vi "FlexMag - 23-03-2023.vi"() -> ()   [LabVIEW 2018] (continued)
                      frame False {
                        n9835 = local write "trns 3-4 led 3"(TRUE ("trns 1-2 led 1")) -> ()
                        n9836 = Wait (ms)(milliseconds to wait=u32 100) -> ()  [unwired: 1 out]
                      }
                      frame True {
                      }
                    }
                  }
                }
              }
              frame #9 {
                n9837 = local read "ch3-4 transfer"() -> (w15268:bool)
                n9838 = case shown="True" w15268 {
                  frame False {
                  }
                  frame True {
                    n9839 = local read "ABORT"() -> (w15269:bool)
                    n9840 = case shown="False" w15269 {
                      frame False {
                        n9841 = while {
                          i -> [w15274]
                          stop <- w15275 stop-if-true
                          n9842 = Greater Or Equal?(x=w15274, y=100) -> (x >= y?=w15272:bool)
                          n9843 = case shown="True" w15272 {
                            frame False {
                            }
                            frame True {
                              n9844 = local write "trns error"(TRUE ("TRNS error")) -> ()
                              n9845 = local write "Warning Message"("Transfer process canceled!\nCH3 TGV Control Problem" ("Warning Message")) -> ()
                            }
                          }
                          n9846 = local read "CH3_TGV_Control_DI"() -> (w15271:bool)
                          n9847 = case shown="True" w15271 {
                            tunnel: [TRUE ("CH1_Trns_BP_Left_DO") FALSE ("CH1_Trns_BP_Left_DO")] -> w15270
                            frame False {
                            }
                            frame True {
                              n9848 = Wait Until Next ms Multiple(millisecond multiple=u32 200) -> ()  [unwired: 1 out]
                              n9849 = local write "CH3_TGV_Control_DO"(FALSE ("CH1_Trns_BP_Left_DO")) -> ()
                            }
                          }
                          n9850 = local read "ch3-4 transfer"() -> (w15278:bool)
                          n9851 = local read "ABORT"() -> (w15277:bool)
                          n9852 = Not(x=w15278) -> (.not. x?=w15276:bool)
                          n9853 = Compound Arithmetic op=OR(w15270, w15277, w15276) -> (w15275:bool)
                        }
                      }
                      frame True {
                      }
                    }
                  }
                }
              }
              frame #10 {
                n9854 = local read "ch3-4 transfer"() -> (w15285:bool)
                n9855 = case shown="True" w15285 {
                  frame False {
                  }
                  frame True {
                    n9856 = local read "ABORT"() -> (w15286:bool)
                    n9857 = case shown="False" w15286 {
                      frame False {
                        n9858 = local write "trns 3-4 led 4"(TRUE ("trns 1-2 led 1")) -> ()
                        n9859 = Wait (ms)(milliseconds to wait=u32 100) -> ()  [unwired: 1 out]
                      }
                      frame True {
                      }
                    }
                  }
                }
              }
              frame #11 {
                n9860 = local read "ch3-4 transfer"() -> (w15289:bool)
                n9861 = case shown="True" w15289 {
                  frame False {
                  }
                  frame True {
                    n9862 = local read "ABORT"() -> (w15290:bool)
                    n9863 = case shown="False" w15290 {
                      frame False {
                        n9864 = while {
                          i -> [w15295]
                          stop <- w15296 stop-if-true
                          n9865 = local read "CH1_Trns_Interlock_DI"() -> (w15291:bool)
                          n9866 = Greater Or Equal?(x=w15295, y=100) -> (x >= y?=w15293:bool)
                          n9867 = case shown="True" w15293 {
                            frame False {
                            }
                            frame True {
                              n9868 = local write "Warning Message"("Transfer process canceled!\nCH1 Interlock problem" ("Warning Message")) -> ()
                              n9869 = local write "trns error"(TRUE ("TRNS error")) -> ()
                            }
                          }
                          n9870 = case shown="False" w15291 {
                            tunnel: [w15300 TRUE ("CH1_Trns_BP_Left_DO")] -> w15292
                            frame False {
                              n9871 = local read "CH1_TGV_Control_DI"() -> (w15301:bool)
                              n9872 = case shown="False" w15301 {
                                tunnel: [FALSE ("CH1_Trns_BP_Left_DO") TRUE ("CH1_Trns_BP_Left_DO")] -> w15300
                                frame False {
                                n9873 = Wait Until Next ms Multiple(millisecond multiple=u32 200) -> ()  [unwired: 1 out]
                                n9874 = local write "CH1_TGV_Control_DO"(TRUE ("CH1_Trns_BP_Left_DO")) -> ()
                                }
                                frame True {
                                }
                              }
                            }
                            frame True {
                            }
                          }
                          n9875 = local read "ch3-4 transfer"() -> (w15299:bool)
                          n9876 = local read "ABORT"() -> (w15298:bool)
                          n9877 = Not(x=w15299) -> (.not. x?=w15297:bool)
                          n9878 = Compound Arithmetic op=OR(w15292, w15298, w15297) -> (w15296:bool)
                        }
                      }
                      frame True {
                      }
                    }
                  }
                }
              }
              frame #12 {
                n9879 = local read "ch3-4 transfer"() -> (w15309:bool)
                n9880 = case shown="True" w15309 {
                  frame False {
                  }
                  frame True {
                    n9881 = local read "ABORT"() -> (w15310:bool)
                    n9882 = case shown="False" w15310 {
                      frame False {
                        w15311 = TRUE ("CH3_Right_Limit_DO")
                        n9883 = local write "trns 3-4 led 5"(TRUE ("trns 1-2 led 1")) -> ()
                        n9884 = Wait (ms)(milliseconds to wait=u32 100) -> ()  [unwired: 1 out]
                        n9885 = local write "CH3_Right_Limit_DO"(w15311) -> ()
                        n9886 = local write "CH3_Right_Slow_DO"(w15311) -> ()
                        n9887 = local write "CH3_Left_Slow_DO"(w15311) -> ()
                        n9888 = local write "CH3_Left_Limit_DO"(w15311) -> ()
                      }
                      frame True {
                      }
                    }
                  }
                }
              }
              frame #13 {
                n9889 = local read "ch3-4 transfer"() -> (w15314:bool)
                n9890 = case shown="True" w15314 {
                  frame False {
                  }
                  frame True {
                    n9891 = local read "ABORT"() -> (w15315:bool)
                    n9892 = case shown="False" w15315 {
                      frame False {
                        n9893 = while {
                          i -> [w15320]
                          stop <- w15321 stop-if-true
                          n9894 = local read "CH2_Trns_Interlock_DI"() -> (w15316:bool)
                          n9895 = Greater Or Equal?(x=w15320, y=100) -> (x >= y?=w15318:bool)
                          n9896 = case shown="True" w15318 {
                            frame False {
                            }
                            frame True {
                              n9897 = local write "Warning Message"("Transfer process canceled!\nCH2 Interlock problem" ("Warning Message")) -> ()
                              n9898 = local write "trns error"(TRUE ("TRNS error")) -> ()
                            }
                          }
                          n9899 = case shown="False" w15316 {
                            tunnel: [w15325 TRUE ("CH1_Trns_BP_Left_DO")] -> w15317
                            frame False {
                              n9900 = local read "CH2_TGV_Control_DI"() -> (w15326:bool)
                              n9901 = case shown="False" w15326 {
                                tunnel: [FALSE ("CH1_Trns_BP_Left_DO") TRUE ("CH1_Trns_BP_Left_DO")] -> w15325
                                frame False {
                                n9902 = Wait Until Next ms Multiple(millisecond multiple=u32 200) -> ()  [unwired: 1 out]
                                n9903 = local write "CH2_TGV_Control_DO"(TRUE ("CH1_Trns_BP_Left_DO")) -> ()
                                }
                                frame True {
                                }
                              }
                            }
                            frame True {
                            }
                          }
                          n9904 = local read "ch3-4 transfer"() -> (w15324:bool)
                          n9905 = local read "ABORT"() -> (w15323:bool)
                          n9906 = Not(x=w15324) -> (.not. x?=w15322:bool)
                          n9907 = Compound Arithmetic op=OR(w15317, w15323, w15322) -> (w15321:bool)
                        }
                      }
                      frame True {
                      }
                    }
                  }
                }
              }
              frame #14 {
                n9908 = local read "ch3-4 transfer"() -> (w15334:bool)
                n9909 = case shown="True" w15334 {
                  frame False {
                  }
                  frame True {
                    n9910 = local read "ABORT"() -> (w15335:bool)
                    n9911 = case shown="False" w15335 {
                      frame False {
                        n9912 = local write "trns 3-4 led 6"(TRUE ("trns 1-2 led 1")) -> ()
                        n9913 = Wait (ms)(milliseconds to wait=u32 100) -> ()  [unwired: 1 out]
                      }
                      frame True {
                      }
                    }
                  }
                }
              }
              frame #15 {
                n9914 = local read "ch3-4 transfer"() -> (w15338:bool)
                n9915 = case shown="True" w15338 {
                  frame False {
                  }
                  frame True {
                    n9916 = local read "ABORT"() -> (w15339:bool)
                    n9917 = case shown="False" w15339 {
                      frame False {
                        n9918 = while {
                          i -> [w15344]
                          stop <- w15345 stop-if-true
                          n9919 = local read "CH4_Trns_Interlock_DI"() -> (w15340:bool)
                          n9920 = Greater Or Equal?(x=w15344, y=100) -> (x >= y?=w15342:bool)
                          n9921 = case shown="True" w15342 {
                            frame False {
                            }
                            frame True {
                              n9922 = local write "Warning Message"("Transfer process canceled!\nCH4 Interlock problem" ("Warning Message")) -> ()
                              n9923 = local write "trns error"(TRUE ("TRNS error")) -> ()
                            }
                          }
                          n9924 = case shown="False" w15340 {
                            tunnel: [w15349 TRUE ("CH1_Trns_BP_Left_DO")] -> w15341
                            frame False {
                              n9925 = local read "CH4_TGV_Control_DI"() -> (w15350:bool)
                              n9926 = case shown="False" w15350 {
                                tunnel: [FALSE ("CH1_Trns_BP_Left_DO") TRUE ("CH1_Trns_BP_Left_DO")] -> w15349
                                frame False {
                                n9927 = Wait Until Next ms Multiple(millisecond multiple=u32 200) -> ()  [unwired: 1 out]
                                n9928 = local write "CH4_TGV_Control_DO"(TRUE ("CH1_Trns_BP_Left_DO")) -> ()
                                }
                                frame True {
                                }
                              }
                            }
                            frame True {
                            }
                          }
                          n9929 = local read "ch3-4 transfer"() -> (w15348:bool)
                          n9930 = local read "ABORT"() -> (w15347:bool)
                          n9931 = Not(x=w15348) -> (.not. x?=w15346:bool)
                          n9932 = Compound Arithmetic op=OR(w15341, w15347, w15346) -> (w15345:bool)
                        }
                      }
                      frame True {
                      }
                    }
                  }
                }
              }
              frame #16 {
                n9933 = local read "ch3-4 transfer"() -> (w15358:bool)
                n9934 = case shown="True" w15358 {
                  frame False {
                  }
                  frame True {
                    n9935 = local read "ABORT"() -> (w15359:bool)
                    n9936 = case shown="False" w15359 {
                      frame False {
                        n9937 = local write "trns 3-4 led 7"(TRUE ("trns 1-2 led 1")) -> ()
                        n9938 = Wait (ms)(milliseconds to wait=u32 100) -> ()  [unwired: 1 out]
                      }
                      frame True {
                      }
                    }
                  }
                }
              }
              frame #17 {
                n9939 = local read "ch3-4 transfer"() -> (w15362:bool)
                n9940 = case shown="True" w15362 {
                  frame False {
                  }
                  frame True {
                    n9941 = local read "ABORT"() -> (w15363:bool)
                    n9942 = case shown="False" w15363 {
                      frame False {
                        n9943 = while {
                          i -> [w15367]
                          stop <- w15368 stop-if-true
                          n9944 = Greater Or Equal?(x=w15367, y=100) -> (x >= y?=w15365:bool)
                          n9945 = case shown="True" w15365 {
                            frame False {
                            }
                            frame True {
                              n9946 = local write "Warning Message"("Transfer process canceled!\nRight Slow Sensor problem" ("Warning Message")) -> ()
                              n9947 = local write "trns error"(TRUE ("TRNS error")) -> ()
                            }
                          }
                          n9948 = disable-structure shown="Enabled" {
                            disable-tunnel: [w15373 w15378] -> w15364
                            frame Disabled {
                              n9949 = local read "Cnt_Right_Slow DI"() -> (w15372:bool)
                              n9950 = case shown="False" w15372 {
                                tunnel: [FALSE ("CH1_Trns_BP_Left_DO") TRUE ("CH1_Trns_BP_Left_DO")] -> w15373
                                frame False {
                                n9951 = Wait Until Next ms Multiple(millisecond multiple=u32 200) -> ()  [unwired: 1 out]
                                n9952 = local write "Cnt_Right_Slow DO"(TRUE ("CH1_Trns_BP_Left_DO")) -> ()
                                }
                                frame True {
                                }
                              }
                            }
                            frame Enabled {
                              n9953 = local read "CH3_Right_Slow_DI"() -> (w15379:bool)
                              n9954 = case shown="True" w15379 {
                                tunnel: [TRUE FALSE] -> w15378
                                frame False {
                                }
                                frame True {
                                n9955 = Wait Until Next ms Multiple(millisecond multiple=u32 200) -> ()  [unwired: 1 out]
                                n9956 = local write "CH3_Right_Slow_DO"(TRUE ("CH2_Right_Limit_DO")) -> ()
                                }
                              }
                            }
                          }
                          n9957 = local read "ch3-4 transfer"() -> (w15371:bool)
                          n9958 = local read "ABORT"() -> (w15370:bool)
                          n9959 = Not(x=w15371) -> (.not. x?=w15369:bool)
                          n9960 = Compound Arithmetic op=OR(w15364, w15370, w15369) -> (w15368:bool)
                        }
                      }
                      frame True {
                      }
                    }
                  }
                }
              }
              frame #18 {
                n9961 = local read "ch3-4 transfer"() -> (w15386:bool)
                n9962 = case shown="True" w15386 {
                  frame False {
                  }
                  frame True {
                    n9963 = local read "ABORT"() -> (w15387:bool)
                    n9964 = case shown="False" w15387 {
                      frame False {
                        n9965 = local write "trns 3-4 led 8"(TRUE ("trns 1-2 led 1")) -> ()
                        n9966 = Wait (ms)(milliseconds to wait=u32 100) -> ()  [unwired: 1 out]
                      }
                      frame True {
                      }
                    }
                  }
                }
              }
              frame #19 {
                n9967 = local read "ch3-4 transfer"() -> (w15390:bool)
                n9968 = case shown="True" w15390 {
                  frame False {
                  }
                  frame True {
                    n9969 = local read "ABORT"() -> (w15391:bool)
                    n9970 = case shown="False" w15391 {
                      frame False {
                        n9971 = while {
                          i -> [w15395]
                          stop <- w15396 stop-if-true
                          n9972 = Greater Or Equal?(x=w15395, y=100) -> (x >= y?=w15393:bool)
                          n9973 = case shown="True" w15393 {
                            frame False {
                            }
                            frame True {
                              n9974 = local write "Warning Message"("Transfer process canceled!\nRight Limit Sensor problem" ("Warning Message")) -> ()
                              n9975 = local write "trns error"(TRUE ("TRNS error")) -> ()
                            }
                          }
                          n9976 = disable-structure shown="Enabled" {
                            disable-tunnel: [w15401 w15406] -> w15392
                            frame Disabled {
                              n9977 = local read "Cnt_Right_Limit DI"() -> (w15400:bool)
                              n9978 = case shown="False" w15400 {
                                tunnel: [FALSE ("CH1_Trns_BP_Left_DO") TRUE ("CH1_Trns_BP_Left_DO")] -> w15401
                                frame False {
                                n9979 = Wait Until Next ms Multiple(millisecond multiple=u32 200) -> ()  [unwired: 1 out]
                                n9980 = local write "Cnt_Right_Limit DO"(TRUE ("CH1_Trns_BP_Left_DO")) -> ()
                                }
                                frame True {
                                }
                              }
                            }
                            frame Enabled {
                              n9981 = local read "CH3_Right_Limit_DI"() -> (w15407:bool)
                              n9982 = case shown="True" w15407 {
                                tunnel: [TRUE FALSE] -> w15406
                                frame False {
                                }
                                frame True {
                                n9983 = Wait Until Next ms Multiple(millisecond multiple=u32 200) -> ()  [unwired: 1 out]
                                n9984 = local write "CH3_Right_Limit_DO"(TRUE ("CH2_Right_Limit_DO")) -> ()
                                }
                              }
                            }
                          }
                          n9985 = local read "ch3-4 transfer"() -> (w15399:bool)
                          n9986 = local read "ABORT"() -> (w15398:bool)
                          n9987 = Not(x=w15399) -> (.not. x?=w15397:bool)
                          n9988 = Compound Arithmetic op=OR(w15392, w15398, w15397) -> (w15396:bool)
                        }
                      }
                      frame True {
                      }
                    }
                  }
                }
              }
              frame #20 {
                n9989 = local read "ch3-4 transfer"() -> (w15414:bool)
                n9990 = case shown="True" w15414 {
                  frame False {
                  }
                  frame True {
                    n9991 = local read "ABORT"() -> (w15415:bool)
                    n9992 = case shown="False" w15415 {
                      frame False {
                        n9993 = local write "trns 3-4 led 9"(TRUE ("trns 1-2 led 1")) -> ()
                        n9994 = Wait (ms)(milliseconds to wait=u32 100) -> ()  [unwired: 1 out]
                      }
                      frame True {
                      }
                    }
                  }
                }
              }
              frame #21 {
                n9995 = local read "ch3-4 transfer"() -> (w15418:bool)
                n9996 = case shown="True" w15418 {
                  frame False {
                  }
                  frame True {
                    n9997 = local read "ABORT"() -> (w15419:bool)
                    n9998 = case shown="False" w15419 {
                      frame False {
                        n9999 = while {
                          i -> [w15423]
                          stop <- w15424 stop-if-true
                          n10000 = Greater Or Equal?(x=w15423, y=100) -> (x >= y?=w15421:bool)
                          n10001 = case shown="True" w15421 {
                            frame False {
                            }
                            frame True {
                              n10002 = local write "Warning Message"("Transfer process canceled!\nLeft Slow Sensor problem" ("Warning Message")) -> ()
                              n10003 = local write "trns error"(TRUE ("TRNS error")) -> ()
                            }
                          }
                          n10004 = disable-structure shown="Enabled" {
                            disable-tunnel: [w15429 w15434] -> w15420
                            frame Disabled {
                              n10005 = local read "Cnt_Left_Slow DI"() -> (w15428:bool)
                              n10006 = case shown="False" w15428 {
                                tunnel: [FALSE ("CH1_Trns_BP_Left_DO") TRUE ("CH1_Trns_BP_Left_DO")] -> w15429
                                frame False {
                                n10007 = Wait Until Next ms Multiple(millisecond multiple=u32 200) -> ()  [unwired: 1 out]
                                n10008 = local write "Cnt_Left_Slow DO"(TRUE ("CH1_Trns_BP_Left_DO")) -> ()
                                }
                                frame True {
                                }
                              }
                            }
                            frame Enabled {
                              n10009 = local read "CH3_Left_Slow_DI"() -> (w15435:bool)
                              n10010 = case shown="True" w15435 {
                                tunnel: [TRUE FALSE] -> w15434
                                frame False {
                                }
                                frame True {
                                n10011 = Wait Until Next ms Multiple(millisecond multiple=u32 200) -> ()  [unwired: 1 out]
                                n10012 = local write "CH3_Left_Slow_DO"(TRUE ("CH2_Right_Limit_DO")) -> ()
                                }
                              }
                            }
                          }
                          n10013 = local read "ch3-4 transfer"() -> (w15427:bool)
                          n10014 = local read "ABORT"() -> (w15426:bool)
                          n10015 = Not(x=w15427) -> (.not. x?=w15425:bool)
                          n10016 = Compound Arithmetic op=OR(w15420, w15426, w15425) -> (w15424:bool)
                        }
                      }
                      frame True {
                      }
                    }
                  }
                }
              }
              frame #22 {
                n10017 = local read "ch3-4 transfer"() -> (w15442:bool)
                n10018 = case shown="True" w15442 {
                  frame False {
                  }
                  frame True {
                    n10019 = local read "ABORT"() -> (w15443:bool)
                    n10020 = case shown="False" w15443 {
                      frame False {
                        n10021 = local write "trns 3-4 led 10"(TRUE ("trns 1-2 led 1")) -> ()
                        n10022 = Wait (ms)(milliseconds to wait=u32 100) -> ()  [unwired: 1 out]
                      }
                      frame True {
                      }
                    }
                  }
                }
              }
              frame #23 {
                n10023 = local read "ch3-4 transfer"() -> (w15446:bool)
                n10024 = case shown="True" w15446 {
                  frame False {
                  }
                  frame True {
                    n10025 = local read "ABORT"() -> (w15447:bool)
                    n10026 = case shown="False" w15447 {
                      frame False {
                        n10027 = while {
                          i -> [w15451]
                          stop <- w15452 stop-if-true
                          n10028 = Greater Or Equal?(x=w15451, y=100) -> (x >= y?=w15449:bool)
                          n10029 = case shown="True" w15449 {
                            frame False {
                            }
                            frame True {
                              n10030 = local write "Warning Message"("Transfer process canceled!\nLeft Limit Sensor problem" ("Warning Message")) -> ()
                              n10031 = local write "trns error"(TRUE ("TRNS error")) -> ()
                            }
                          }
                          n10032 = disable-structure shown="Enabled" {
                            disable-tunnel: [w15457 w15462] -> w15448
                            frame Disabled {
                              n10033 = local read "Cnt_Left_Limit DI"() -> (w15456:bool)
                              n10034 = case shown="False" w15456 {
                                tunnel: [FALSE ("CH1_Trns_BP_Left_DO") TRUE ("CH1_Trns_BP_Left_DO")] -> w15457
                                frame False {
                                n10035 = Wait Until Next ms Multiple(millisecond multiple=u32 200) -> ()  [unwired: 1 out]
                                n10036 = local write "Cnt_Left_Limit DO"(TRUE ("CH1_Trns_BP_Left_DO")) -> ()
                                }
                                frame True {
                                }
                              }
                            }
                            frame Enabled {
                              n10037 = local read "CH3_Left_Limit_DI"() -> (w15463:bool)
                              n10038 = case shown="True" w15463 {
                                tunnel: [TRUE FALSE] -> w15462
                                frame False {
                                }
                                frame True {
                                n10039 = Wait Until Next ms Multiple(millisecond multiple=u32 200) -> ()  [unwired: 1 out]
                                n10040 = local write "CH3_Left_Limit_DO"(TRUE ("CH2_Right_Limit_DO")) -> ()
                                }
                              }
                            }
                          }
                          n10041 = local read "ch3-4 transfer"() -> (w15455:bool)
                          n10042 = local read "ABORT"() -> (w15454:bool)
                          n10043 = Not(x=w15455) -> (.not. x?=w15453:bool)
                          n10044 = Compound Arithmetic op=OR(w15448, w15454, w15453) -> (w15452:bool)
                        }
                      }
                      frame True {
                      }
                    }
                  }
                }
              }
              frame #24 {
                n10045 = local read "ch3-4 transfer"() -> (w15470:bool)
                n10046 = case shown="True" w15470 {
                  frame False {
                  }
                  frame True {
                    n10047 = local read "ABORT"() -> (w15471:bool)
                    n10048 = case shown="False" w15471 {
                      frame False {
                        n10049 = local write "trns 3-4 led 11"(TRUE ("trns 1-2 led 1")) -> ()
                        n10050 = Wait (ms)(milliseconds to wait=u32 100) -> ()  [unwired: 1 out]
                      }
                      frame True {
                      }
                    }
                  }
                }
              }
              frame #25 {
                n10051 = local read "ch3-4 transfer"() -> (w15474:bool)
                n10052 = case shown="True" w15474 {
                  frame False {
                  }
                  frame True {
                    n10053 = local read "ABORT"() -> (w15475:bool)
                    n10054 = case shown="False" w15475 {
                      frame False {
                        w15476 = FALSE ("CH4_SRV1_Piston_For_DO")
                        n10055 = local write "CH4_Left_Limit_DO"(w15476) -> ()
                        n10056 = local write "CH4_Left_Slow_DO"(w15476) -> ()
                        n10057 = Wait (ms)(milliseconds to wait=u32 2000) -> ()  [unwired: 1 out]
                      }
                      frame True {
                      }
                    }
                  }
                }
              }
              frame #26 {
                n10058 = local read "ch3-4 transfer"() -> (w15478:bool)
                n10059 = case shown="True" w15478 {
                  frame False {
                  }
                  frame True {
                    n10060 = local read "ABORT"() -> (w15479:bool)
                    n10061 = case shown="False" w15479 {
                      frame False {
                        n10062 = while {
                          i -> [w15484]
                          stop <- w15485 stop-if-true
                          n10063 = Greater Or Equal?(x=w15484, y=100) -> (x >= y?=w15482:bool)
                          n10064 = case shown="True" w15482 {
                            frame False {
                            }
                            frame True {
                              n10065 = local write "Warning Message"("Transfer process canceled!\nCassette Servo Direction problem" ("Warning Message")) -> ()
                              n10066 = local write "trns error"(TRUE ("TRNS error")) -> ()
                            }
                          }
                          n10067 = local read "Casette_Servo_Left_Direction DI"() -> (w15480:bool)
                          n10068 = case shown="False" w15480 {
                            tunnel: [FALSE ("CH1_Trns_BP_Left_DO") TRUE ("CH1_Trns_BP_Left_DO")] -> w15481
                            frame False {
                              n10069 = local write "Casette_Servo_Left_Direction DO"(TRUE ("CH1_Trns_BP_Left_DO")) -> ()
                              n10070 = Wait Until Next ms Multiple(millisecond multiple=u32 200) -> ()  [unwired: 1 out]
                            }
                            frame True {
                            }
                          }
                          n10071 = local read "ch3-4 transfer"() -> (w15488:bool)
                          n10072 = local read "ABORT"() -> (w15487:bool)
                          n10073 = Not(x=w15488) -> (.not. x?=w15486:bool)
                          n10074 = Compound Arithmetic op=OR(w15481, w15487, w15486) -> (w15485:bool)
                        }
                      }
                      frame True {
                      }
                    }
                  }
                }
              }
              frame #27 {
                n10075 = local read "ch3-4 transfer"() -> (w15495:bool)
                n10076 = case shown="True" w15495 {
                  frame False {
                  }
                  frame True {
                    n10077 = local read "ABORT"() -> (w15496:bool)
                    n10078 = case shown="False" w15496 {
                      frame False {
                        n10079 = local write "trns 3-4 led 12"(TRUE ("trns 1-2 led 1")) -> ()
                        n10080 = Wait (ms)(milliseconds to wait=u32 100) -> ()  [unwired: 1 out]
                      }
                      frame True {
                      }
                    }
                  }
                }
              }
              frame #28 {
                n10081 = local read "ch3-4 transfer"() -> (w15499:bool)
                n10082 = case shown="True" w15499 {
                  frame False {
                  }
                  frame True {
                    n10083 = local read "ABORT"() -> (w15500:bool)
                    n10084 = case shown="False" w15500 {
                      frame False {
                        n10085 = stacked-sequence {
                          frame #0 {
                            n10086 = local read "Cst_Speed_High"() -> (w15501:dbl)
                            n10087 = Wait (ms)(milliseconds to wait=u32 100) -> ()  [unwired: 1 out]
                            n10088 = local write "Cassette_Servo_Speed AO"(w15501) -> ()
                          }
                          frame #1 {
                            n10089 = Wait (ms)(milliseconds to wait=u32 200) -> ()  [unwired: 1 out]
                          }
                          frame #2 {
                            n10090 = local write "Cassette_Servo_Speed Set"(TRUE ("Cassette_Servo_Speed Set")) -> ()
                          }
                          frame #3 {
                            n10091 = Wait (ms)(milliseconds to wait=u32 300) -> ()  [unwired: 1 out]
                          }
                        }
                      }
                      frame True {
                      }
                    }
                  }
                }
              }
              frame #29 {
                n10092 = local read "ch3-4 transfer"() -> (w15506:bool)
                n10093 = case shown="True" w15506 {
                  frame False {
                  }
                  frame True {
                    n10094 = local read "ABORT"() -> (w15507:bool)
                    n10095 = case shown="False" w15507 {
                      frame False {
                        n10096 = local write "trns 3-4 led 13"(TRUE ("trns 1-2 led 1")) -> ()
                        n10097 = Wait (ms)(milliseconds to wait=u32 100) -> ()  [unwired: 1 out]
                      }
                      frame True {
                      }
                    }
                  }
                }
              }
              frame #30 {
                n10098 = local read "ch3-4 transfer"() -> (w15510:bool)
                n10099 = case shown="True" w15510 {
                  frame False {
                  }
                  frame True {
                    n10100 = local read "ABORT"() -> (w15511:bool)
                    n10101 = case shown="False" w15511 {
                      frame False {
                        n10102 = while {
                          i -> [w15516]
                          stop <- w15517 stop-if-true
                          n10103 = Greater Or Equal?(x=w15516, y=100) -> (x >= y?=w15514:bool)
                          n10104 = case shown="True" w15514 {
                            frame False {
                            }
                            frame True {
                              n10105 = local write "Warning Message"("Transfer process canceled!\nCassette Servo Start problem" ("Warning Message")) -> ()
                              n10106 = local write "trns error"(TRUE ("TRNS error")) -> ()
                            }
                          }
                          n10107 = local read "Casette_Servo_Start/Stop DI"() -> (w15512:bool)
                          n10108 = case shown="False" w15512 {
                            tunnel: [FALSE ("CH1_Trns_BP_Left_DO") TRUE ("CH1_Trns_BP_Left_DO")] -> w15513
                            frame False {
                              n10109 = local write "Casette_Servo_Start/Stop DO"(TRUE ("CH1_Trns_BP_Left_DO")) -> ()
                              n10110 = Wait Until Next ms Multiple(millisecond multiple=u32 200) -> ()  [unwired: 1 out]
                            }
                            frame True {
                            }
                          }
                          n10111 = local read "ch3-4 transfer"() -> (w15520:bool)
                          n10112 = local read "ABORT"() -> (w15519:bool)
                          n10113 = Not(x=w15520) -> (.not. x?=w15518:bool)
                          n10114 = Compound Arithmetic op=OR(w15513, w15519, w15518) -> (w15517:bool)
                        }
                      }
                      frame True {
                      }
                    }
                  }
                }
              }
              frame #31 {
                n10115 = local read "ch3-4 transfer"() -> (w15527:bool)
                n10116 = case shown="True" w15527 {
                  frame False {
                  }
                  frame True {
                    n10117 = local read "ABORT"() -> (w15528:bool)
                    n10118 = case shown="False" w15528 {
                      frame False {
                        n10119 = local write "trns 3-4 led 14"(TRUE ("trns 1-2 led 1")) -> ()
                        n10120 = Wait (ms)(milliseconds to wait=u32 100) -> ()  [unwired: 1 out]
                      }
                      frame True {
                      }
                    }
                  }
                }
              }
              frame #32 {
                n10121 = local read "ch3-4 transfer"() -> (w15531:bool)
                n10122 = case shown="True" w15531 {
                  frame False {
                  }
                  frame True {
                    n10123 = local read "ABORT"() -> (w15532:bool)
                    n10124 = case shown="False" w15532 {
                      frame False {
                        n10125 = disable-structure shown="Disabled" {
                          frame Disabled {
                            n10126 = stacked-sequence {
                              frame #0 {
                                n10127 = while {
                                i -> [w15539]
                                stop <- w15540 stop-if-true
                                n10128 = Greater Or Equal?(x=w15539, y=1500) -> (x >= y?=w15537:bool)
                                n10129 = case shown="True" w15537 {
                                frame False {
                                }
                                frame True {
                                n10130 = local write "Warning Message"("Transfer process canceled!\nCounter problem" ("Warning Message")) -> ()
                                n10131 = local write "trns error"(TRUE ("TRNS error")) -> ()
                                }
                                }
                                n10132 = local read "Counter Read Data"() -> (w15535:i16)
                                n10133 = Greater Or Equal?(x=w15535, y=i16 5820) -> (x >= y?=w15533:bool)
                                n10134 = case shown="True" w15533 {
                                tunnel: [FALSE ("CH1_Trns_BP_Left_DO") TRUE ("CH1_Trns_BP_Left_DO")] -> w15536
                                frame False {
                                n10135 = Wait Until Next ms Multiple(millisecond multiple=u32 200) -> ()  [unwired: 1 out]
                                }
                                frame True {
                                }
                                }
                                n10136 = local read "ch3-4 transfer"() -> (w15543:bool)
                                n10137 = local read "ABORT"() -> (w15542:bool)
                                n10138 = Not(x=w15543) -> (.not. x?=w15541:bool)
                                n10139 = Compound Arithmetic op=OR(w15536, w15542, w15541) -> (w15540:bool)
                                }
                              }
                              frame #1 {
                                n10140 = while {
                                i -> [w15553]
                                stop <- w15554 stop-if-true
                                n10141 = Greater Or Equal?(x=w15553, y=100) -> (x >= y?=w15551:bool)
                                n10142 = case shown="True" w15551 {
                                frame False {
                                }
                                frame True {
                                n10143 = local write "Warning Message"("Transfer process canceled!\nLeft Slow Sensor problem" ("Warning Message")) -> ()
                                n10144 = local write "trns error"(TRUE ("TRNS error")) -> ()
                                }
                                }
                                n10145 = local read "Cnt_Left_Slow DI"() -> (w15549:bool)
                                n10146 = case shown="True" w15549 {
                                tunnel: [TRUE ("CH1_Trns_BP_Left_DO") FALSE ("CH1_Trns_BP_Left_DO")] -> w15550
                                frame False {
                                }
                                frame True {
                                n10147 = Wait Until Next ms Multiple(millisecond multiple=u32 200) -> ()  [unwired: 1 out]
                                n10148 = local write "Cnt_Left_Slow DO"(FALSE ("TRNS error")) -> ()
                                }
                                }
                                n10149 = local read "ch3-4 transfer"() -> (w15557:bool)
                                n10150 = local read "ABORT"() -> (w15556:bool)
                                n10151 = Not(x=w15557) -> (.not. x?=w15555:bool)
                                n10152 = Compound Arithmetic op=OR(w15550, w15556, w15555) -> (w15554:bool)
                                }
                              }
                              frame #2 {
                                n10153 = while {
                                i -> [w15568]
                                stop <- w15569 stop-if-true
                                n10154 = Greater Or Equal?(x=w15568, y=100) -> (x >= y?=w15566:bool)
                                n10155 = case shown="True" w15566 {
                                frame False {
                                }
                                frame True {
                                n10156 = local write "Warning Message"("Transfer process canceled!\nLeft Limit Sensor problem" ("Warning Message")) -> ()
                                n10157 = local write "trns error"(TRUE ("TRNS error")) -> ()
                                }
                                }
                                n10158 = local read "Cnt_Left_Limit DI"() -> (w15564:bool)
                                n10159 = case shown="True" w15564 {
                                tunnel: [TRUE ("CH1_Trns_BP_Left_DO") FALSE ("CH1_Trns_BP_Left_DO")] -> w15565
                                frame False {
                                }
                                frame True {
                                n10160 = Wait Until Next ms Multiple(millisecond multiple=u32 200) -> ()  [unwired: 1 out]
                                n10161 = local write "Cnt_Left_Limit DO"(FALSE ("TRNS error")) -> ()
                                }
                                }
                                n10162 = local read "ch3-4 transfer"() -> (w15572:bool)
                                n10163 = local read "ABORT"() -> (w15571:bool)
                                n10164 = Not(x=w15572) -> (.not. x?=w15570:bool)
                                n10165 = Compound Arithmetic op=OR(w15565, w15571, w15570) -> (w15569:bool)
                                }
                              }
                            }
                          }
                          frame Enabled {
                          }
                        }
                      }
                      frame True {
                      }
                    }
                  }
                }
              }
              frame #33 {
                n10166 = local read "ch3-4 transfer"() -> (w15579:bool)
                n10167 = case shown="True" w15579 {
                  frame False {
                  }
                  frame True {
                    n10168 = local read "ABORT"() -> (w15580:bool)
                    n10169 = case shown="False" w15580 {
                      frame False {
                        n10170 = local write "trns 3-4 led 15"(TRUE ("trns 1-2 led 1")) -> ()
                        n10171 = Wait (ms)(milliseconds to wait=u32 100) -> ()  [unwired: 1 out]
                      }
                      frame True {
                      }
                    }
                  }
                }
              }
              frame #34 {
                n10172 = local read "ch3-4 transfer"() -> (w15583:bool)
                n10173 = case shown="True" w15583 {
                  frame False {
                  }
                  frame True {
                    n10174 = local read "ABORT"() -> (w15584:bool)
                    n10175 = case shown="False" w15584 {
                      frame False {
                        n10176 = stacked-sequence {
                          frame #0 {
                            n10177 = while {
                              i -> [w15589]
                              stop <- w15590 stop-if-true
                              n10178 = Greater Or Equal?(x=w15589, y=1500) -> (x >= y?=w15587:bool)
                              n10179 = case shown="True" w15587 {
                                frame False {
                                }
                                frame True {
                                n10180 = local write "Warning Message"("Transfer process canceled!\nCH4 Left Slow Sensor problem" ("Warning Message")) -> ()
                                n10181 = local write "trns error"(TRUE ("TRNS error")) -> ()
                                }
                              }
                              n10182 = local read "CH4_Left_Slow_DI"() -> (w15585:bool)
                              n10183 = case shown="True" w15585 {
                                tunnel: [FALSE ("CH1_Trns_BP_Left_DO") TRUE ("CH1_Trns_BP_Left_DO")] -> w15586
                                frame False {
                                n10184 = Wait Until Next ms Multiple(millisecond multiple=u32 200) -> ()  [unwired: 1 out]
                                }
                                frame True {
                                }
                              }
                              n10185 = local read "ch3-4 transfer"() -> (w15593:bool)
                              n10186 = local read "ABORT"() -> (w15592:bool)
                              n10187 = Not(x=w15593) -> (.not. x?=w15591:bool)
                              n10188 = Compound Arithmetic op=OR(w15586, w15592, w15591) -> (w15590:bool)
                            }
                          }
                          frame #1 {
                            n10189 = flat-sequence {
                              frame #0 {
                                n10190 = local read "Cst_Speed_Low"() -> (w15599:dbl)
                                n10191 = local write "Cassette_Servo_Speed AO"(w15599) -> ()
                                n10192 = Wait (ms)(milliseconds to wait=u32 100) -> ()  [unwired: 1 out]
                              }
                              frame #1 {
                                n10193 = local write "Cassette_Servo_Speed Set"(TRUE ("Cassette_Servo_Speed Set")) -> ()
                              }
                              frame #2 {
                                n10194 = Wait (ms)(milliseconds to wait=u32 100) -> ()  [unwired: 1 out]
                              }
                            }
                          }
                          frame #2 {
                            n10195 = while {
                              i -> [w15606]
                              stop <- w15607 stop-if-true
                              n10196 = Greater Or Equal?(x=w15606, y=100) -> (x >= y?=w15604:bool)
                              n10197 = case shown="True" w15604 {
                                frame False {
                                }
                                frame True {
                                n10198 = local write "Warning Message"("Transfer process canceled!\nLeft Slow Sensor problem" ("Warning Message")) -> ()
                                n10199 = local write "trns error"(TRUE ("TRNS error")) -> ()
                                }
                              }
                              n10200 = disable-structure shown="Enabled" {
                                disable-tunnel: [w15612 w15617] -> w15603
                                frame Disabled {
                                n10201 = local read "Cnt_Left_Slow DI"() -> (w15611:bool)
                                n10202 = case shown="False" w15611 {
                                tunnel: [FALSE ("CH1_Trns_BP_Left_DO") TRUE ("CH1_Trns_BP_Left_DO")] -> w15612
                                frame False {
                                n10203 = Wait Until Next ms Multiple(millisecond multiple=u32 200) -> ()  [unwired: 1 out]
                                n10204 = local write "Cnt_Left_Slow DO"(TRUE ("TRNS error")) -> ()
                                }
                                frame True {
                                }
                                }
                                }
                                frame Enabled {
                                n10205 = local read "CH4_Left_Slow_DI"() -> (w15618:bool)
                                n10206 = case shown="True" w15618 {
                                tunnel: [TRUE FALSE] -> w15617
                                frame False {
                                }
                                frame True {
                                n10207 = Wait Until Next ms Multiple(millisecond multiple=u32 200) -> ()  [unwired: 1 out]
                                n10208 = local write "CH4_Left_Slow_DO"(TRUE ("CH2_Right_Limit_DO")) -> ()
                                }
                                }
                                }
                              }
                              n10209 = local read "ch3-4 transfer"() -> (w15610:bool)
                              n10210 = local read "ABORT"() -> (w15609:bool)
                              n10211 = Not(x=w15610) -> (.not. x?=w15608:bool)
                              n10212 = Compound Arithmetic op=OR(w15603, w15609, w15608) -> (w15607:bool)
                            }
                          }
                        }
                      }
                      frame True {
                      }
                    }
                  }
                }
              }
              frame #35 {
                n10213 = local read "ch3-4 transfer"() -> (w15625:bool)
                n10214 = case shown="True" w15625 {
                  frame False {
                  }
                  frame True {
                    n10215 = local read "ABORT"() -> (w15626:bool)
                    n10216 = case shown="False" w15626 {
                      frame False {
                        n10217 = local write "trns 3-4 led 16"(TRUE ("trns 1-2 led 1")) -> ()
                        n10218 = Wait (ms)(milliseconds to wait=u32 100) -> ()  [unwired: 1 out]
                      }
                      frame True {
                      }
                    }
                  }
                }
              }
              frame #36 {
                n10219 = local read "ch3-4 transfer"() -> (w15629:bool)
                n10220 = case shown="True" w15629 {
                  frame False {
                  }
                  frame True {
                    n10221 = local read "ABORT"() -> (w15630:bool)
                    n10222 = case shown="False" w15630 {
                      frame False {
                        n10223 = stacked-sequence {
                          frame #0 {
                            n10224 = while {
                              i -> [w15635]
                              stop <- w15636 stop-if-true
                              n10225 = Greater Or Equal?(x=w15635, y=600) -> (x >= y?=w15633:bool)
                              n10226 = case shown="True" w15633 {
                                frame False {
                                }
                                frame True {
                                n10227 = local write "Warning Message"("Transfer process canceled!\nCH4 Left Limit Sensor problem" ("Warning Message")) -> ()
                                n10228 = local write "trns error"(TRUE ("TRNS error")) -> ()
                                }
                              }
                              n10229 = local read "CH4_Left_Limit_DI"() -> (w15631:bool)
                              n10230 = case shown="True" w15631 {
                                tunnel: [FALSE ("CH1_Trns_BP_Left_DO") TRUE ("CH1_Trns_BP_Left_DO")] -> w15632
                                frame False {
                                n10231 = Wait Until Next ms Multiple(millisecond multiple=u32 200) -> ()  [unwired: 1 out]
                                }
                                frame True {
                                }
                              }
                              n10232 = local read "ch3-4 transfer"() -> (w15639:bool)
                              n10233 = local read "ABORT"() -> (w15638:bool)
                              n10234 = Not(x=w15639) -> (.not. x?=w15637:bool)
                              n10235 = Compound Arithmetic op=OR(w15632, w15638, w15637) -> (w15636:bool)
                            }
                          }
                          frame #1 {
                            n10236 = while {
                              i -> [w15649]
                              stop <- w15650 stop-if-true
                              n10237 = Greater Or Equal?(x=w15649, y=100) -> (x >= y?=w15647:bool)
                              n10238 = case shown="True" w15647 {
                                frame False {
                                }
                                frame True {
                                n10239 = local write "Warning Message"("Transfer process canceled!\nCassette Servo couldn't be stopped" ("Warning Message")) -> ()
                                n10240 = local write "trns error"(TRUE ("TRNS error")) -> ()
                                }
                              }
                              n10241 = local read "Casette_Servo_Start/Stop DI"() -> (w15645:bool)
                              n10242 = case shown="True" w15645 {
                                tunnel: [TRUE ("CH1_Trns_BP_Left_DO") FALSE ("CH1_Trns_BP_Left_DO")] -> w15646
                                frame False {
                                }
                                frame True {
                                n10243 = Wait Until Next ms Multiple(millisecond multiple=u32 200) -> ()  [unwired: 1 out]
                                n10244 = local write "Casette_Servo_Start/Stop DO"(FALSE ("TRNS error")) -> ()
                                }
                              }
                              n10245 = local read "ch3-4 transfer"() -> (w15653:bool)